vi "Dresden R2R Sputter 03.02.2018 IY24.vi"() -> ()   [LabVIEW 2009] (continued)
          }
        }
        n1372 = case shown="0, Default" w2342 {
          tunnel: w2348 -> [_ w2692 _]
          tunnel: w2349 -> [_ _ w2693]
          tunnel: [u32[][] [] ("24-bit pixmap") w2692 w2693] -> w2341
          frame #0 {
          }
          frame #1 {
          }
          frame #2 {
          }
        }
        n1373 = case shown="0, Default" w2339 {
          tunnel: w2348 -> [_ w2689 _]
          tunnel: w2349 -> [_ _ w2690]
          tunnel: [u32[][] [] ("24-bit pixmap") w2689 w2690] -> w2340
          frame #0 {
          }
          frame #1 {
          }
          frame #2 {
          }
        }
        n1374 = case shown="0, Default" w2327 {
          tunnel: w2348 -> [_ w2686 _]
          tunnel: w2349 -> [_ _ w2687]
          tunnel: [u32[][] [] ("24-bit pixmap") w2686 w2687] -> w2326
          frame #0 {
          }
          frame #1 {
          }
          frame #2 {
          }
        }
        n1375 = case shown="0, Default" w2323 {
          tunnel: w2348 -> [_ w2683 _]
          tunnel: w2349 -> [_ _ w2684]
          tunnel: [u32[][] [] ("24-bit pixmap") w2683 w2684] -> w2324
          frame #0 {
          }
          frame #1 {
          }
          frame #2 {
          }
        }
        n1376 = case shown="3" w2290 {
          tunnel: w2284 -> [_ w2679 _ _]
          tunnel: w2283 -> [_ _ w2680 _]
          tunnel: [u32[][] [] ("24-bit pixmap") w2679 w2680 w2681] -> w2291
          tunnel: w1979 -> [_ _ _ w2681]
          frame #0 {
          }
          frame #1 {
          }
          frame #2 {
          }
          frame #3 {
          }
        }
        n1377 = case shown="3" w2293 {
          tunnel: w2284 -> [_ w2675 _ _]
          tunnel: w2283 -> [_ _ w2676 _]
          tunnel: [u32[][] [] ("24-bit pixmap") w2675 w2676 w2677] -> w2292
          tunnel: w1979 -> [_ _ _ w2677]
          frame #0 {
          }
          frame #1 {
          }
          frame #2 {
          }
          frame #3 {
          }
        }
        n1378 = case shown="3" w2305 {
          tunnel: w2284 -> [_ w2671 _ _]
          tunnel: w2283 -> [_ _ w2672 _]
          tunnel: [u32[][] [] ("24-bit pixmap") w2671 w2672 w2673] -> w2306
          tunnel: w1979 -> [_ _ _ w2673]
          frame #0 {
          }
          frame #1 {
          }
          frame #2 {
          }
          frame #3 {
          }
        }
        n1379 = case shown="3" w2309 {
          tunnel: w2284 -> [_ w2667 _ _]
          tunnel: w2283 -> [_ _ w2668 _]
          tunnel: [u32[][] [] ("24-bit pixmap") w2667 w2668 w2669] -> w2308
          tunnel: w1979 -> [_ _ _ w2669]
          frame #0 {
          }
          frame #1 {
          }
          frame #2 {
          }
          frame #3 {
          }
        }
        n1380 = case shown="2" w2274 {
          tunnel: w2280 -> [_ w2664 _]
          tunnel: w2281 -> [_ _ w2665]
          tunnel: [u32[][] [] ("24-bit pixmap") w2664 w2665] -> w2273
          frame #0 {
          }
          frame #1 {
          }
          frame #2 {
          }
        }
        n1381 = case shown="2" w2271 {
          tunnel: w2280 -> [_ w2661 _]
          tunnel: w2281 -> [_ _ w2662]
          tunnel: [u32[][] [] ("24-bit pixmap") w2661 w2662] -> w2272
          frame #0 {
          }
          frame #1 {
          }
          frame #2 {
          }
        }
        n1382 = case shown="2" w2259 {
          tunnel: w2280 -> [_ w2658 _]
          tunnel: w2281 -> [_ _ w2659]
          tunnel: [u32[][] [] ("24-bit pixmap") w2658 w2659] -> w2258
          frame #0 {
          }
          frame #1 {
          }
          frame #2 {
          }
        }
        n1383 = case shown="2" w2255 {
          tunnel: w2280 -> [_ w2655 _]
          tunnel: w2281 -> [_ _ w2656]
          tunnel: [u32[][] [] ("24-bit pixmap") w2655 w2656] -> w2256
          frame #0 {
          }
          frame #1 {
          }
          frame #2 {
          }
        }
        n1384 = case shown="0, Default" w2222 {
          tunnel: w2216 -> [_ w2652 _]
          tunnel: w2215 -> [_ _ w2653]
          tunnel: [u32[][] [] ("24-bit pixmap") w2652 w2653] -> w2223
          frame #0 {
          }
          frame #1 {
          }
          frame #2 {
          }
        }
        n1385 = case shown="0, Default" w2225 {
          tunnel: w2216 -> [_ w2649 _]
          tunnel: w2215 -> [_ _ w2650]
          tunnel: [u32[][] [] ("24-bit pixmap") w2649 w2650] -> w2224
          frame #0 {
          }
          frame #1 {
          }
          frame #2 {
          }
        }
        n1386 = case shown="0, Default" w2237 {
          tunnel: w2216 -> [_ w2646 _]
          tunnel: w2215 -> [_ _ w2647]
          tunnel: [u32[][] [] ("24-bit pixmap") w2646 w2647] -> w2238
          frame #0 {
          }
          frame #1 {
          }
          frame #2 {
          }
        }
        n1387 = case shown="0, Default" w2241 {
          tunnel: w2216 -> [_ w2643 _]
          tunnel: w2215 -> [_ _ w2644]
          tunnel: [u32[][] [] ("24-bit pixmap") w2643 w2644] -> w2240
          frame #0 {
          }
          frame #1 {
          }
          frame #2 {
          }
        }
        n1388 = case shown="0, Default" w2206 {
          tunnel: w2212 -> [_ w2640 _]
          tunnel: w2213 -> [_ _ w2641]
          tunnel: [u32[][] [] ("24-bit pixmap") w2640 w2641] -> w2205
          frame #0 {
          }
          frame #1 {
          }
          frame #2 {
          }
        }
        n1389 = case shown="0, Default" w2203 {
          tunnel: w2212 -> [_ w2637 _]
          tunnel: w2213 -> [_ _ w2638]
          tunnel: [u32[][] [] ("24-bit pixmap") w2637 w2638] -> w2204
          frame #0 {
          }
          frame #1 {
          }
          frame #2 {
          }
        }
        n1390 = case shown="0, Default" w2191 {
          tunnel: w2212 -> [_ w2634 _]
          tunnel: w2213 -> [_ _ w2635]
          tunnel: [u32[][] [] ("24-bit pixmap") w2634 w2635] -> w2190
          frame #0 {
          }
          frame #1 {
          }
          frame #2 {
          }
        }
        n1391 = case shown="0, Default" w2154 {
          tunnel: w2148 -> [_ w2628 _]
          tunnel: w2147 -> [_ _ w2629]
          tunnel: [u32[][] [] ("24-bit pixmap") w2628 w2629] -> w2155
          frame #0 {
          }
          frame #1 {
          }
          frame #2 {
          }
        }
        n1392 = case shown="0, Default" w2187 {
          tunnel: w2212 -> [_ w2631 _]
          tunnel: w2213 -> [_ _ w2632]
          tunnel: [u32[][] [] ("24-bit pixmap") w2631 w2632] -> w2188
          frame #0 {
          }
          frame #1 {
          }
          frame #2 {
          }
        }
        n1393 = case shown="0, Default" w2157 {
          tunnel: w2148 -> [_ w2625 _]
          tunnel: w2147 -> [_ _ w2626]
          tunnel: [u32[][] [] ("24-bit pixmap") w2625 w2626] -> w2156
          frame #0 {
          }
          frame #1 {
          }
          frame #2 {
          }
        }
        n1394 = case shown="0, Default" w2169 {
          tunnel: w2148 -> [_ w2622 _]
          tunnel: w2147 -> [_ _ w2623]
          tunnel: [u32[][] [] ("24-bit pixmap") w2622 w2623] -> w2170
          frame #0 {
          }
          frame #1 {
          }
          frame #2 {
          }
        }
        n1395 = case shown="0, Default" w2141 {
          tunnel: w2066 -> [_ w2616 _]
          tunnel: w2118 -> [_ _ w2617]
          tunnel: [u32[][] [] ("24-bit pixmap") w2616 w2617] -> w2144
          frame #0 {
          }
          frame #1 {
          }
          frame #2 {
          }
        }
        n1396 = case shown="2" w2173 {
          tunnel: w2148 -> [_ w2619 _]
          tunnel: w2147 -> [_ _ w2620]
          tunnel: [u32[][] [] ("24-bit pixmap") w2619 w2620] -> w2172
          frame #0 {
          }
          frame #1 {
          }
          frame #2 {
          }
        }
        n1397 = case shown="2" w2131 {
          tunnel: w2066 -> [_ w2613 _]
          tunnel: w2118 -> [_ _ w2614]
          tunnel: [u32[][] [] ("24-bit pixmap") w2613 w2614] -> w2117
          frame #0 {
          }
          frame #1 {
          }
          frame #2 {
          }
        }
        n1398 = case shown="1" w2130 {
          tunnel: w2066 -> [_ w2610 _]
          tunnel: w2118 -> [_ _ w2611]
          tunnel: [u32[][] [] ("24-bit pixmap") w2610 w2611] -> w2116
          frame #0 {
          }
          frame #1 {
          }
          frame #2 {
          }
        }
        n1399 = case shown="2" w2129 {
          tunnel: w2066 -> [_ w2607 _]
          tunnel: w2118 -> [_ _ w2608]
          tunnel: [u32[][] [] ("24-bit pixmap") w2607 w2608] -> w2115
          frame #0 {
          }
          frame #1 {
          }
          frame #2 {
          }
        }
        n1400 = case shown="2" w2113 {
          tunnel: w2065 -> [_ w2604 _]
          tunnel: w2064 -> [_ _ w2605]
          tunnel: [u32[][] [] ("24-bit pixmap") w2604 w2605] -> w2114
          frame #0 {
          }
          frame #1 {
          }
          frame #2 {
          }
        }
        n1401 = case shown="2" w2108 {
          tunnel: w2065 -> [_ w2601 _]
          tunnel: w2064 -> [_ _ w2602]
          tunnel: [u32[][] [] ("24-bit pixmap") w2601 w2602] -> w2107
          frame #0 {
          }
          frame #1 {
          }
          frame #2 {
          }
        }
        n1402 = case shown="2" w2105 {
          tunnel: w2065 -> [_ w2598 _]
          tunnel: w2064 -> [_ _ w2599]
          tunnel: [u32[][] [] ("24-bit pixmap") w2598 w2599] -> w2106
          frame #0 {
          }
          frame #1 {
          }
          frame #2 {
          }
        }
        n1403 = case shown="2" w2100 {
          tunnel: w2063 -> [_ w2595 _]
          tunnel: w2062 -> [_ _ w2596]
          tunnel: [u32[][] [] ("24-bit pixmap") w2595 w2596] -> w2099
          frame #0 {
          }
          frame #1 {
          }
          frame #2 {
          }
        }
        n1404 = case shown="2" w2092 {
          tunnel: w2063 -> [_ w2589 _]
          tunnel: w2062 -> [_ _ w2590]
          tunnel: [u32[][] [] ("24-bit pixmap") w2589 w2590] -> w2091
          frame #0 {
          }
          frame #1 {
          }
          frame #2 {
          }
        }
        n1405 = case shown="2" w2097 {
          tunnel: w2063 -> [_ w2592 _]
          tunnel: w2062 -> [_ _ w2593]
          tunnel: [u32[][] [] ("24-bit pixmap") w2592 w2593] -> w2098
          frame #0 {
          }
          frame #1 {
          }
          frame #2 {
          }
        }
        n1406 = case shown="2" w2060 {
          tunnel: w2037 -> [_ w2586 _]
          tunnel: w2036 -> [_ _ w2587]
          tunnel: [u32[][] [] ("24-bit pixmap") w2586 w2587] -> w2061
          frame #0 {
          }
          frame #1 {
          }
          frame #2 {
          }
        }
        n1407 = case shown="2" w2055 {
          tunnel: w2037 -> [_ w2583 _]
          tunnel: w2036 -> [_ _ w2584]
          tunnel: [u32[][] [] ("24-bit pixmap") w2583 w2584] -> w2054
          frame #0 {
          }
          frame #1 {
          }
          frame #2 {
          }
        }
        n1408 = case shown="2" w2052 {
          tunnel: w2037 -> [_ w2580 _]
          tunnel: w2036 -> [_ _ w2581]
          tunnel: [u32[][] [] ("24-bit pixmap") w2580 w2581] -> w2053
          frame #0 {
          }
          frame #1 {
          }
          frame #2 {
          }
        }
        n1409 = case shown="2" w2033 {
          tunnel: w1989 -> [_ w2577 _]
          tunnel: w1988 -> [_ _ w2578]
          tunnel: [u32[][] [] ("24-bit pixmap") w2577 w2578] -> w2032
          frame #0 {
          }
          frame #1 {
          }
          frame #2 {
          }
        }
        n1410 = case shown="2" w2030 {
          tunnel: w1989 -> [_ w2574 _]
          tunnel: w1988 -> [_ _ w2575]
          tunnel: [u32[][] [] ("24-bit pixmap") w2574 w2575] -> w2031
          frame #0 {
          }
          frame #1 {
          }
          frame #2 {
          }
        }
        n1411 = case shown="2" w2025 {
          tunnel: w1989 -> [_ w2571 _]
          tunnel: w1988 -> [_ _ w2572]
          tunnel: [u32[][] [] ("24-bit pixmap") w2571 w2572] -> w2024
          frame #0 {
          }
          frame #1 {
          }
          frame #2 {
          }
        }
        n1412 = case shown="2" w2022 {
          tunnel: w1987 -> [_ w2568 _]
          tunnel: w1986 -> [_ _ w2569]
          tunnel: [u32[][] [] ("24-bit pixmap") w2568 w2569] -> w2023
          frame #0 {
          }
          frame #1 {
          }
          frame #2 {
          }
        }
        n1413 = case shown="2" w2017 {
          tunnel: w1987 -> [_ w2565 _]
          tunnel: w1986 -> [_ _ w2566]
          tunnel: [u32[][] [] ("24-bit pixmap") w2565 w2566] -> w2016
          frame #0 {
          }
          frame #1 {
          }
          frame #2 {
          }
        }
        n1414 = case shown="0, Default" w2014 {
          tunnel: w1987 -> [_ w2562 _]
          tunnel: w1986 -> [_ _ w2563]
          tunnel: [u32[][] [] ("24-bit pixmap") w2562 w2563] -> w2015
          frame #0 {
          }
          frame #1 {
          }
          frame #2 {
          }
        }
        n1415 = case shown="1" w1974 {
          tunnel: w1947 -> [_ w2560]
          tunnel: [u32[][] [] ("24-bit pixmap") w2560] -> w1971
          frame #0 {
          }
          frame #1 {
          }
        }
        n1416 = case shown="1" w1968 {
          tunnel: w1947 -> [_ w2558]
          tunnel: [u32[][] [] ("24-bit pixmap") w2558] -> w1970
          frame #0 {
          }
          frame #1 {
          }
        }
        n1417 = case shown="1" w1958 {
          tunnel: w1947 -> [_ w2556]
          tunnel: [u32[][] [] ("24-bit pixmap") w2556] -> w1956
          frame #0 {
          }
          frame #1 {
          }
        }
        n1418 = case shown="1" w1952 {
          tunnel: w1947 -> [_ w2554]
          tunnel: [u32[][] [] ("24-bit pixmap") w2554] -> w1954
          frame #0 {
          }
          frame #1 {
          }
        }
        n1419 = call-poly <vilib>:"Draw Unflattened Pixmap.vi"("data (RGB format)"=w1941) -> ("new picture"=w2546:picture)  [unwired: 8 in]
        n1420 = call-poly <vilib>:"Draw Unflattened Pixmap.vi"("picture"=w2546, "top left point(0, 0)"=cluster{"x":i16, "y":i16} {"x"=1103, "y"=31}, "data (RGB format)"=w2545) -> ("new picture"=w2537:picture)  [unwired: 6 in]
        n1421 = call-poly <vilib>:"Draw Unflattened Pixmap.vi"("picture"=w2537, "top left point(0, 0)"=cluster{"x":i16, "y":i16} {"x"=778, "y"=31}, "data (RGB format)"=w2544) -> ("new picture"=w2529:picture)  [unwired: 6 in]
        n1422 = call-poly <vilib>:"Draw Unflattened Pixmap.vi"("picture"=w2529, "top left point(0, 0)"=cluster{"x":i16, "y":i16} {"x"=453, "y"=31}, "data (RGB format)"=w2530) -> ("new picture"=w1940:picture)  [unwired: 6 in]
        n1423 = call-poly <vilib>:"Draw Unflattened Pixmap.vi"("picture"=w1940, "top left point(0, 0)"=cluster{"x":i16, "y":i16} {"x"=128, "y"=31}, "data (RGB format)"=w2528) -> ("new picture"=w2490:picture)  [unwired: 6 in]
        n1424 = call-poly <vilib>:"Draw Unflattened Pixmap.vi"("picture"=w2490, "top left point(0, 0)"=cluster{"x":i16, "y":i16} {"x"=1076, "y"=146} ("top left point(0, 0) 4"), "data (RGB format)"=w2497) -> ("new picture"=w2505:picture)  [unwired: 6 in]
        n1425 = call-poly <vilib>:"Draw Unflattened Pixmap.vi"("picture"=w2505, "top left point(0, 0)"=cluster{"x":i16, "y":i16} {"x"=751, "y"=146} ("top left point(0, 0) 3"), "data (RGB format)"=w2498) -> ("new picture"=w2513:picture)  [unwired: 6 in]
        n1426 = call-poly <vilib>:"Draw Unflattened Pixmap.vi"("picture"=w2513, "top left point(0, 0)"=cluster{"x":i16, "y":i16} {"x"=426, "y"=146} ("top left point(0, 0) 2"), "data (RGB format)"=w2512) -> ("new picture"=w2521:picture)  [unwired: 6 in]
        n1427 = call-poly <vilib>:"Draw Unflattened Pixmap.vi"("picture"=w2521, "top left point(0, 0)"=cluster{"x":i16, "y":i16} {"x"=100, "y"=146}, "data (RGB format)"=w2514) -> ("new picture"=w2452:picture)  [unwired: 6 in]
        n1428 = call-poly <vilib>:"Draw Unflattened Pixmap.vi"("picture"=w2452, "top left point(0, 0)"=cluster{"x":i16, "y":i16} {"x"=1181, "y"=150} ("top left point(0, 0) 4"), "data (RGB format)"=w2477) -> ("new picture"=w2469:picture)  [unwired: 6 in]
        n1429 = call-poly <vilib>:"Draw Unflattened Pixmap.vi"("picture"=w2469, "top left point(0, 0)"=cluster{"x":i16, "y":i16} {"x"=856, "y"=150} ("top left point(0, 0) 3"), "data (RGB format)"=w2476) -> ("new picture"=w2461:picture)  [unwired: 6 in]
        n1430 = call-poly <vilib>:"Draw Unflattened Pixmap.vi"("picture"=w2461, "top left point(0, 0)"=cluster{"x":i16, "y":i16} {"x"=531, "y"=150} ("top left point(0, 0) 2"), "data (RGB format)"=w2462) -> ("new picture"=w2453:picture)  [unwired: 6 in]
        n1431 = call-poly <vilib>:"Draw Unflattened Pixmap.vi"("picture"=w2453, "top left point(0, 0)"=cluster{"x":i16, "y":i16} {"x"=205, "y"=150}, "data (RGB format)"=w2460) -> ("new picture"=w2418:picture)  [unwired: 6 in]
        n1432 = call-poly <vilib>:"Draw Unflattened Pixmap.vi"("picture"=w2418, "top left point(0, 0)"=cluster{"x":i16, "y":i16} {"x"=1162, "y"=215} ("top left point(0, 0) 4"), "data (RGB format)"=w2427) -> ("new picture"=w2435:picture)  [unwired: 6 in]
        n1433 = call-poly <vilib>:"Draw Unflattened Pixmap.vi"("picture"=w2435, "top left point(0, 0)"=cluster{"x":i16, "y":i16} {"x"=838, "y"=215} ("top left point(0, 0) 3"), "data (RGB format)"=w2428) -> ("new picture"=w2443:picture)  [unwired: 6 in]
        n1434 = call-poly <vilib>:"Draw Unflattened Pixmap.vi"("picture"=w2443, "top left point(0, 0)"=cluster{"x":i16, "y":i16} {"x"=513, "y"=217} ("top left point(0, 0) 2"), "data (RGB format)"=w2442) -> ("new picture"=w2451:picture)  [unwired: 6 in]
        n1435 = call-poly <vilib>:"Draw Unflattened Pixmap.vi"("picture"=w2451, "top left point(0, 0)"=cluster{"x":i16, "y":i16} {"x"=187, "y"=215}, "data (RGB format)"=w2444) -> ("new picture"=w2384:picture)  [unwired: 6 in]
        n1436 = call-poly <vilib>:"Draw Unflattened Pixmap.vi"("picture"=w2384, "top left point(0, 0)"=cluster{"x":i16, "y":i16} {"x"=1120, "y"=323} ("top left point(0, 0) 4"), "data (RGB format)"=w2409) -> ("new picture"=w2401:picture)  [unwired: 6 in]
        n1437 = call-poly <vilib>:"Draw Unflattened Pixmap.vi"("picture"=w2401, "top left point(0, 0)"=cluster{"x":i16, "y":i16} {"x"=794, "y"=323} ("top left point(0, 0) 3"), "data (RGB format)"=w2408) -> ("new picture"=w2393:picture)  [unwired: 6 in]
        n1438 = call-poly <vilib>:"Draw Unflattened Pixmap.vi"("picture"=w2393, "top left point(0, 0)"=cluster{"x":i16, "y":i16} {"x"=468, "y"=323} ("top left point(0, 0) 2"), "data (RGB format)"=w2394) -> ("new picture"=w2385:picture)  [unwired: 6 in]
        n1439 = call-poly <vilib>:"Draw Unflattened Pixmap.vi"("picture"=w2385, "top left point(0, 0)"=cluster{"x":i16, "y":i16} {"x"=143, "y"=323}, "data (RGB format)"=w2392) -> ("new picture"=w2350:picture)  [unwired: 6 in]
        n1440 = call-poly <vilib>:"Draw Unflattened Pixmap.vi"("picture"=w2350, "top left point(0, 0)"=cluster{"x":i16, "y":i16} {"x"=1061, "y"=399} ("top left point(0, 0) 4"), "data (RGB format)"=w2359) -> ("new picture"=w2367:picture)  [unwired: 6 in]
        n1441 = call-poly <vilib>:"Draw Unflattened Pixmap.vi"("picture"=w2367, "top left point(0, 0)"=cluster{"x":i16, "y":i16} {"x"=735, "y"=399} ("top left point(0, 0) 3"), "data (RGB format)"=w2360) -> ("new picture"=w2375:picture)  [unwired: 6 in]
        n1442 = call-poly <vilib>:"Draw Unflattened Pixmap.vi"("picture"=w2375, "top left point(0, 0)"=cluster{"x":i16, "y":i16} {"x"=409, "y"=399} ("top left point(0, 0) 2"), "data (RGB format)"=w2374) -> ("new picture"=w2383:picture)  [unwired: 6 in]
        n1443 = call-poly <vilib>:"Draw Unflattened Pixmap.vi"("picture"=w2383, "top left point(0, 0)"=cluster{"x":i16, "y":i16} {"x"=83, "y"=399}, "data (RGB format)"=w2376) -> ("new picture"=w2316:picture)  [unwired: 6 in]
        n1444 = call-poly <vilib>:"Draw Unflattened Pixmap.vi"("picture"=w2316, "top left point(0, 0)"=cluster{"x":i16, "y":i16} {"x"=1117, "y"=399} ("top left point(0, 0) 4"), "data (RGB format)"=w2341) -> ("new picture"=w2333:picture)  [unwired: 6 in]
        n1445 = call-poly <vilib>:"Draw Unflattened Pixmap.vi"("picture"=w2333, "top left point(0, 0)"=cluster{"x":i16, "y":i16} {"x"=791, "y"=399} ("top left point(0, 0) 3"), "data (RGB format)"=w2340) -> ("new picture"=w2325:picture)  [unwired: 6 in]
        n1446 = call-poly <vilib>:"Draw Unflattened Pixmap.vi"("picture"=w2325, "top left point(0, 0)"=cluster{"x":i16, "y":i16} {"x"=465, "y"=399} ("top left point(0, 0) 2"), "data (RGB format)"=w2326) -> ("new picture"=w2317:picture)  [unwired: 6 in]
        n1447 = call-poly <vilib>:"Draw Unflattened Pixmap.vi"("picture"=w2317, "top left point(0, 0)"=cluster{"x":i16, "y":i16} {"x"=139, "y"=398}, "data (RGB format)"=w2324) -> ("new picture"=w2282:picture)  [unwired: 6 in]
        n1448 = call-poly <vilib>:"Draw Unflattened Pixmap.vi"("picture"=w2282, "top left point(0, 0)"=cluster{"x":i16, "y":i16} {"x"=1109, "y"=459} ("top left point(0, 0) 4"), "data (RGB format)"=w2291) -> ("new picture"=w2299:picture)  [unwired: 6 in]
        n1449 = call-poly <vilib>:"Draw Unflattened Pixmap.vi"("picture"=w2299, "top left point(0, 0)"=cluster{"x":i16, "y":i16} {"x"=783, "y"=459} ("top left point(0, 0) 3"), "data (RGB format)"=w2292) -> ("new picture"=w2307:picture)  [unwired: 6 in]
        n1450 = call-poly <vilib>:"Draw Unflattened Pixmap.vi"("picture"=w2307, "top left point(0, 0)"=cluster{"x":i16, "y":i16} {"x"=457, "y"=459} ("top left point(0, 0) 2"), "data (RGB format)"=w2306) -> ("new picture"=w2315:picture)  [unwired: 6 in]
        n1451 = call-poly <vilib>:"Draw Unflattened Pixmap.vi"("picture"=w2315, "top left point(0, 0)"=cluster{"x":i16, "y":i16} {"x"=131, "y"=459}, "data (RGB format)"=w2308) -> ("new picture"=w2248:picture)  [unwired: 6 in]
        n1452 = call-poly <vilib>:"Draw Unflattened Pixmap.vi"("picture"=w2248, "top left point(0, 0)"=cluster{"x":i16, "y":i16} {"x"=1038, "y"=701} ("top left point(0, 0) 4"), "data (RGB format)"=w2273) -> ("new picture"=w2265:picture)  [unwired: 6 in]
        n1453 = call-poly <vilib>:"Draw Unflattened Pixmap.vi"("picture"=w2265, "top left point(0, 0)"=cluster{"x":i16, "y":i16} {"x"=712, "y"=701} ("top left point(0, 0) 3"), "data (RGB format)"=w2272) -> ("new picture"=w2257:picture)  [unwired: 6 in]
        n1454 = call-poly <vilib>:"Draw Unflattened Pixmap.vi"("picture"=w2257, "top left point(0, 0)"=cluster{"x":i16, "y":i16} {"x"=386, "y"=701} ("top left point(0, 0) 2"), "data (RGB format)"=w2258) -> ("new picture"=w2249:picture)  [unwired: 6 in]
        n1455 = call-poly <vilib>:"Draw Unflattened Pixmap.vi"("picture"=w2249, "top left point(0, 0)"=cluster{"x":i16, "y":i16} {"x"=60, "y"=701}, "data (RGB format)"=w2256) -> ("new picture"=w2214:picture)  [unwired: 6 in]
        n1456 = call-poly <vilib>:"Draw Unflattened Pixmap.vi"("picture"=w2214, "top left point(0, 0)"=cluster{"x":i16, "y":i16} {"x"=1090, "y"=705} ("top left point(0, 0) 4"), "data (RGB format)"=w2223) -> ("new picture"=w2231:picture)  [unwired: 6 in]
        n1457 = call-poly <vilib>:"Draw Unflattened Pixmap.vi"("picture"=w2231, "top left point(0, 0)"=cluster{"x":i16, "y":i16} {"x"=765, "y"=705} ("top left point(0, 0) 3"), "data (RGB format)"=w2224) -> ("new picture"=w2239:picture)  [unwired: 6 in]
        n1458 = call-poly <vilib>:"Draw Unflattened Pixmap.vi"("picture"=w2239, "top left point(0, 0)"=cluster{"x":i16, "y":i16} {"x"=439, "y"=705} ("top left point(0, 0) 2"), "data (RGB format)"=w2238) -> ("new picture"=w2247:picture)  [unwired: 6 in]
        n1459 = call-poly <vilib>:"Draw Unflattened Pixmap.vi"("picture"=w2247, "top left point(0, 0)"=cluster{"x":i16, "y":i16} {"x"=113, "y"=705}, "data (RGB format)"=w2240) -> ("new picture"=w2180:picture)  [unwired: 6 in]
        n1460 = call-poly <vilib>:"Draw Unflattened Pixmap.vi"("picture"=w2180, "top left point(0, 0)"=cluster{"x":i16, "y":i16} {"x"=1152, "y"=717} ("top left point(0, 0) 4"), "data (RGB format)"=w2205) -> ("new picture"=w2197:picture)  [unwired: 6 in]
        n1461 = call-poly <vilib>:"Draw Unflattened Pixmap.vi"("picture"=w2197, "top left point(0, 0)"=cluster{"x":i16, "y":i16} {"x"=827, "y"=717} ("top left point(0, 0) 3"), "data (RGB format)"=w2204) -> ("new picture"=w2189:picture)  [unwired: 6 in]
        n1462 = call-poly <vilib>:"Draw Unflattened Pixmap.vi"("picture"=w2189, "top left point(0, 0)"=cluster{"x":i16, "y":i16} {"x"=501, "y"=717} ("top left point(0, 0) 2"), "data (RGB format)"=w2190) -> ("new picture"=w2181:picture)  [unwired: 6 in]
        n1463 = call-poly <vilib>:"Draw Unflattened Pixmap.vi"("picture"=w2181, "top left point(0, 0)"=cluster{"x":i16, "y":i16} {"x"=175, "y"=717}, "data (RGB format)"=w2188) -> ("new picture"=w2146:picture)  [unwired: 6 in]
        n1464 = call-poly <vilib>:"Draw Unflattened Pixmap.vi"("picture"=w2146, "top left point(0, 0)"=cluster{"x":i16, "y":i16} {"x"=1164, "y"=753} ("top left point(0, 0) 4"), "data (RGB format)"=w2155) -> ("new picture"=w2163:picture)  [unwired: 6 in]
        n1465 = call-poly <vilib>:"Draw Unflattened Pixmap.vi"("picture"=w2163, "top left point(0, 0)"=cluster{"x":i16, "y":i16} {"x"=838, "y"=753} ("top left point(0, 0) 3"), "data (RGB format)"=w2156) -> ("new picture"=w2171:picture)  [unwired: 6 in]
        n1466 = call-poly <vilib>:"Draw Unflattened Pixmap.vi"("picture"=w2171, "top left point(0, 0)"=cluster{"x":i16, "y":i16} {"x"=512, "y"=753} ("top left point(0, 0) 2"), "data (RGB format)"=w2170) -> ("new picture"=w2179:picture)  [unwired: 6 in]
        n1467 = call-poly <vilib>:"Draw Unflattened Pixmap.vi"("picture"=w2179, "top left point(0, 0)"=cluster{"x":i16, "y":i16} {"x"=186, "y"=753}, "data (RGB format)"=w2172) -> ("new picture"=w2145:picture)  [unwired: 6 in]
        n1468 = call-poly <vilib>:"Draw Unflattened Pixmap.vi"("picture"=w2145, "top left point(0, 0)"=cluster{"x":i16, "y":i16} {"x"=1238, "y"=723}, "data (RGB format)"=w2144) -> ("new picture"=w2126:picture)  [unwired: 6 in]
        n1469 = call-poly <vilib>:"Draw Unflattened Pixmap.vi"("picture"=w2126, "top left point(0, 0)"=cluster{"x":i16, "y":i16} {"x"=913, "y"=723}, "data (RGB format)"=w2117) -> ("new picture"=w2127:picture)  [unwired: 6 in]
        n1470 = call-poly <vilib>:"Draw Unflattened Pixmap.vi"("picture"=w2127, "top left point(0, 0)"=cluster{"x":i16, "y":i16} {"x"=587, "y"=723}, "data (RGB format)"=w2116) -> ("new picture"=w2128:picture)  [unwired: 6 in]
        n1471 = call-poly <vilib>:"Draw Unflattened Pixmap.vi"("picture"=w2128, "top left point(0, 0)"=cluster{"x":i16, "y":i16} {"x"=260, "y"=723}, "data (RGB format)"=w2115) -> ("new picture"=w2090:picture)  [unwired: 6 in]
        n1472 = call-poly <vilib>:"Draw Unflattened Pixmap.vi"("picture"=w2090, "top left point(0, 0)"=cluster{"x":i16, "y":i16} {"x"=1039, "y"=465}, "data (RGB format)"=w2114) -> ("new picture"=w2089:picture)  [unwired: 6 in]
        n1473 = call-poly <vilib>:"Draw Unflattened Pixmap.vi"("picture"=w2089, "top left point(0, 0)"=cluster{"x":i16, "y":i16} {"x"=713, "y"=465}, "data (RGB format)"=w2107) -> ("new picture"=w2088:picture)  [unwired: 6 in]
        n1474 = call-poly <vilib>:"Draw Unflattened Pixmap.vi"("picture"=w2088, "top left point(0, 0)"=cluster{"x":i16, "y":i16} {"x"=387, "y"=465}, "data (RGB format)"=w2106) -> ("new picture"=w2087:picture)  [unwired: 6 in]
        n1475 = call-poly <vilib>:"Draw Unflattened Pixmap.vi"("picture"=w2087, "top left point(0, 0)"=cluster{"x":i16, "y":i16} {"x"=883, "y"=467}, "data (RGB format)"=w2099) -> ("new picture"=w2086:picture)  [unwired: 6 in]
        n1476 = call-poly <vilib>:"Draw Unflattened Pixmap.vi"("picture"=w2086, "top left point(0, 0)"=cluster{"x":i16, "y":i16} {"x"=557, "y"=467}, "data (RGB format)"=w2098) -> ("new picture"=w2085:picture)  [unwired: 6 in]
        n1477 = call-poly <vilib>:"Draw Unflattened Pixmap.vi"("picture"=w2085, "top left point(0, 0)"=cluster{"x":i16, "y":i16} {"x"=232, "y"=467}, "data (RGB format)"=w2091) -> ("new picture"=w2039:picture)  [unwired: 6 in]
        n1478 = call-poly <vilib>:"Draw Unflattened Pixmap.vi"("picture"=w2039, "top left point(0, 0)"=cluster{"x":i16, "y":i16} {"x"=958, "y"=528}, "data (RGB format)"=w2061) -> ("new picture"=w2040:picture)  [unwired: 6 in]
        n1479 = call-poly <vilib>:"Draw Unflattened Pixmap.vi"("picture"=w2040, "top left point(0, 0)"=cluster{"x":i16, "y":i16} {"x"=633, "y"=528}, "data (RGB format)"=w2054) -> ("new picture"=w2038:picture)  [unwired: 6 in]
        n1480 = call-poly <vilib>:"Draw Unflattened Pixmap.vi"("picture"=w2038, "top left point(0, 0)"=cluster{"x":i16, "y":i16} {"x"=308, "y"=528}, "data (RGB format)"=w2053) -> ("new picture"=w2006:picture)  [unwired: 6 in]
        n1481 = call-poly <vilib>:"Draw Unflattened Pixmap.vi"("picture"=w2006, "top left point(0, 0)"=cluster{"x":i16, "y":i16} {"x"=985, "y"=263}, "data (RGB format)"=w2032) -> ("new picture"=w2007:picture)  [unwired: 6 in]
        n1482 = call-poly <vilib>:"Draw Unflattened Pixmap.vi"("picture"=w2007, "top left point(0, 0)"=cluster{"x":i16, "y":i16} {"x"=949, "y"=263}, "data (RGB format)"=w2031) -> ("new picture"=w2008:picture)  [unwired: 6 in]
        n1483 = call-poly <vilib>:"Draw Unflattened Pixmap.vi"("picture"=w2008, "top left point(0, 0)"=cluster{"x":i16, "y":i16} {"x"=660, "y"=263}, "data (RGB format)"=w2024) -> ("new picture"=w2009:picture)  [unwired: 6 in]
        n1484 = call-poly <vilib>:"Draw Unflattened Pixmap.vi"("picture"=w2009, "top left point(0, 0)"=cluster{"x":i16, "y":i16} {"x"=624, "y"=263}, "data (RGB format)"=w2023) -> ("new picture"=w2010:picture)  [unwired: 6 in]
        n1485 = call-poly <vilib>:"Draw Unflattened Pixmap.vi"("picture"=w2010, "top left point(0, 0)"=cluster{"x":i16, "y":i16} {"x"=334, "y"=263}, "data (RGB format)"=w2016) -> ("new picture"=w2011:picture)  [unwired: 6 in]
        n1486 = call-poly <vilib>:"Draw Unflattened Pixmap.vi"("picture"=w2011, "top left point(0, 0)"=cluster{"x":i16, "y":i16} {"x"=298, "y"=263}, "data (RGB format)"=w2015) -> ("new picture"=w1972:picture)  [unwired: 6 in]
        n1487 = call-poly <vilib>:"Draw Unflattened Pixmap.vi"("picture"=w1972, "top left point(0, 0)"=cluster{"x":i16, "y":i16} {"x"=58, "y"=545}, "data (RGB format)"=w1971) -> ("new picture"=w1963:picture)  [unwired: 6 in]
        n1488 = call-poly <vilib>:"Draw Unflattened Pixmap.vi"("picture"=w1963, "top left point(0, 0)"=cluster{"x":i16, "y":i16} {"x"=380, "y"=545}, "data (RGB format)"=w1970) -> ("new picture"=w1955:picture)  [unwired: 6 in]
        n1489 = call-poly <vilib>:"Draw Unflattened Pixmap.vi"("picture"=w1955, "top left point(0, 0)"=cluster{"x":i16, "y":i16} {"x"=705, "y"=545}, "data (RGB format)"=w1956) -> ("new picture"=w1946:picture)  [unwired: 6 in]
        n1490 = call-poly <vilib>:"Draw Unflattened Pixmap.vi"("picture"=w1946, "top left point(0, 0)"=cluster{"x":i16, "y":i16} {"x"=1033, "y"=545}, "data (RGB format)"=w1954) -> ("new picture"=w1945:picture)  [unwired: 6 in]
      }
      frame #1 {
        # "67"
        # "66"
        # "65"
        # "64"
        # "63"
        # "62"
        # "61"
        # "60"
        # "59"
        # "58"
        # "57"
        # "56"
        # "55"
        # "54"
        # "53"
        # "52"
        # "51"
        # "50"
        # "49"
        # "48"
        # "47"
        # "46"
        # "45"
        # "44"
        # "43"
        # "42"
        # "41"
        # "40"
        # "39"
        # "38"
        # "37"
        # "36"
        # "35"
        # "34"
        # "33"
        # "32"
        # "31"
        # "30"
        # "29"
        # "28"
        # "27"
        # "26"
        # "25"
        # "24"
        # "23"
        # "22"
        # "21"
        # "20"
        # "19"
        # "18"
        # "17"
        # "16"
        # "15"
        # "14"
        # "13"
        # "12"
        # "11"
        # "10"
        # "9"
        # "8"
        # "7"
        # "6"
        # "5"
        # "4"
        # "3"
        # "2"
        # "1"
        n1491 = property on="Background" class="Pict"() -> ("Mouse"=w3317:T37)  [unwired: 2 in, 2 out]
        n1492 = Unbundle(w3317) -> ("Mouse Position"=w3316:cluster{"X":i32, "Y":i32}, "Mouse Modifiers"=w3455:T38)
        "Mouse Position" <- w3316
        n1493 = Unbundle(w3316) -> ("X"=w2926:i32, "Y"=w2925:i32)
        n1494 = Unbundle(w3455) -> ("Button Down"=w3064:bool)  [unwired: 3 out]
        n1495 = In Range and Coerce(upper limit=197, x=w2925, lower limit=147) -> (In Range?=w3411:bool)  [unwired: 1 out]
        n1496 = In Range and Coerce(upper limit=197, x=w2925, lower limit=147) -> (In Range?=w3400:bool)  [unwired: 1 out]
        n1497 = In Range and Coerce(upper limit=126, x=w2926, lower limit=99) -> (In Range?=w3410:bool)  [unwired: 1 out]
        n1498 = In Range and Coerce(upper limit=774, x=w2926, lower limit=751) -> (In Range?=w3401:bool)  [unwired: 1 out]
        n1499 = In Range and Coerce(upper limit=197, x=w2925, lower limit=147) -> (In Range?=w3414:bool)  [unwired: 1 out]
        n1500 = In Range and Coerce(upper limit=743, x=w2925, lower limit=720) -> (In Range?=w3370:bool)  [unwired: 1 out]
        n1501 = In Range and Coerce(upper limit=197, x=w2925, lower limit=147) -> (In Range?=w3397:bool)  [unwired: 1 out]
        n1502 = In Range and Coerce(upper limit=446, x=w2926, lower limit=426) -> (In Range?=w3415:bool)  [unwired: 1 out]
        n1503 = In Range and Coerce(upper limit=743, x=w2925, lower limit=720) -> (In Range?=w3381:bool)  [unwired: 1 out]
        n1504 = In Range and Coerce(upper limit=213, x=w2926, lower limit=176) -> (In Range?=w3371:bool)  [unwired: 1 out]
        n1505 = In Range and Coerce(upper limit=1099, x=w2926, lower limit=1076) -> (In Range?=w3396:bool)  [unwired: 1 out]
        n1506 = In Range and Coerce(upper limit=863, x=w2926, lower limit=827) -> (In Range?=w3380:bool)  [unwired: 1 out]
        n1507 = In Range and Coerce(upper limit=347, x=w2925, lower limit=326) -> (In Range?=w3340:bool)  [unwired: 1 out]
        n1508 = In Range and Coerce(upper limit=306, x=w2926, lower limit=267) -> (In Range?=w2955:bool)  [unwired: 1 out]
        n1509 = In Range and Coerce(upper limit=758, x=w2925, lower limit=730) -> (In Range?=w2956:bool)  [unwired: 1 out]
        n1510 = In Range and Coerce(upper limit=633, x=w2926, lower limit=591) -> (In Range?=w2958:bool)  [unwired: 1 out]
        n1511 = In Range and Coerce(upper limit=758, x=w2925, lower limit=730) -> (In Range?=w2957:bool)  [unwired: 1 out]
        n1512 = In Range and Coerce(upper limit=961, x=w2926, lower limit=917) -> (In Range?=w2967:bool)  [unwired: 1 out]
        n1513 = In Range and Coerce(upper limit=758, x=w2925, lower limit=730) -> (In Range?=w2968:bool)  [unwired: 1 out]
        n1514 = In Range and Coerce(upper limit=1283, x=w2926, lower limit=1242) -> (In Range?=w2970:bool)  [unwired: 1 out]
        n1515 = In Range and Coerce(upper limit=758, x=w2925, lower limit=730) -> (In Range?=w2969:bool)  [unwired: 1 out]
        n1516 = In Range and Coerce(upper limit=115, x=w2925, lower limit=31) -> (In Range?=w3432:bool)  [unwired: 1 out]
        n1517 = In Range and Coerce(upper limit=743, x=w2925, lower limit=720) -> (In Range?=w3367:bool)  [unwired: 1 out]
        n1518 = In Range and Coerce(upper limit=347, x=w2925, lower limit=326) -> (In Range?=w3329:bool)  [unwired: 1 out]
        n1519 = In Range and Coerce(upper limit=182, x=w2926, lower limit=144) -> (In Range?=w3339:bool)  [unwired: 1 out]
        n1520 = In Range and Coerce(upper limit=450, x=w2925, lower limit=401) -> (In Range?=w3296:bool)  [unwired: 1 out]
        n1521 = In Range and Coerce(upper limit=456, x=w2925, lower limit=392) -> (In Range?=w3273:bool)  [unwired: 1 out]
        n1522 = In Range and Coerce(upper limit=685, x=w2925, lower limit=536) -> (In Range?=w3100:bool)  [unwired: 1 out]
        n1523 = In Range and Coerce(upper limit=751, x=w2925, lower limit=717) -> (In Range?=w3091:bool)  [unwired: 1 out]
        n1524 = In Range and Coerce(upper limit=212, x=w2926, lower limit=188) -> (In Range?=w2998:bool)  [unwired: 1 out]
        n1525 = In Range and Coerce(upper limit=789, x=w2925, lower limit=762) -> (In Range?=w2997:bool)  [unwired: 1 out]
        n1526 = In Range and Coerce(upper limit=538, x=w2926, lower limit=513) -> (In Range?=w2995:bool)  [unwired: 1 out]
        n1527 = In Range and Coerce(upper limit=789, x=w2925, lower limit=762) -> (In Range?=w2996:bool)  [unwired: 1 out]
        n1528 = In Range and Coerce(upper limit=863, x=w2926, lower limit=840) -> (In Range?=w2986:bool)  [unwired: 1 out]
        n1529 = In Range and Coerce(upper limit=789, x=w2925, lower limit=762) -> (In Range?=w2985:bool)  [unwired: 1 out]
        n1530 = In Range and Coerce(upper limit=1191, x=w2926, lower limit=1164) -> (In Range?=w2983:bool)  [unwired: 1 out]
        n1531 = In Range and Coerce(upper limit=789, x=w2925, lower limit=762) -> (In Range?=w2984:bool)  [unwired: 1 out]
        n1532 = In Range and Coerce(upper limit=85, x=w2926, lower limit=60) -> (In Range?=w2946:bool)  [unwired: 1 out]
        n1533 = In Range and Coerce(upper limit=735, x=w2925, lower limit=710) -> (In Range?=w2945:bool)  [unwired: 1 out]
        n1534 = In Range and Coerce(upper limit=408, x=w2926, lower limit=386) -> (In Range?=w2943:bool)  [unwired: 1 out]
        n1535 = In Range and Coerce(upper limit=735, x=w2925, lower limit=710) -> (In Range?=w2944:bool)  [unwired: 1 out]
        n1536 = In Range and Coerce(upper limit=738, x=w2926, lower limit=712) -> (In Range?=w2934:bool)  [unwired: 1 out]
        n1537 = In Range and Coerce(upper limit=735, x=w2925, lower limit=710) -> (In Range?=w2933:bool)  [unwired: 1 out]
        n1538 = In Range and Coerce(upper limit=1064, x=w2926, lower limit=1033) -> (In Range?=w2931:bool)  [unwired: 1 out]
        n1539 = In Range and Coerce(upper limit=735, x=w2925, lower limit=710) -> (In Range?=w2932:bool)  [unwired: 1 out]
        n1540 = In Range and Coerce(upper limit=115, x=w2925, lower limit=31) -> (In Range?=w3444:bool)  [unwired: 1 out]
        n1541 = In Range and Coerce(upper limit=212, x=w2926, lower limit=128) -> (In Range?=w3433:bool)  [unwired: 1 out]
        n1542 = In Range and Coerce(upper limit=742, x=w2925, lower limit=720) -> (In Range?=w3384:bool)  [unwired: 1 out]
        n1543 = In Range and Coerce(upper limit=539, x=w2926, lower limit=503) -> (In Range?=w3366:bool)  [unwired: 1 out]
        n1544 = In Range and Coerce(upper limit=832, x=w2926, lower limit=795) -> (In Range?=w3330:bool)  [unwired: 1 out]
        n1545 = In Range and Coerce(upper limit=450, x=w2925, lower limit=401) -> (In Range?=w3307:bool)  [unwired: 1 out]
        n1546 = In Range and Coerce(upper limit=107, x=w2926, lower limit=85) -> (In Range?=w3297:bool)  [unwired: 1 out]
        n1547 = In Range and Coerce(upper limit=456, x=w2925, lower limit=392) -> (In Range?=w3262:bool)  [unwired: 1 out]
        n1548 = In Range and Coerce(upper limit=211, x=w2926, lower limit=129) -> (In Range?=w3272:bool)  [unwired: 1 out]
        n1549 = In Range and Coerce(upper limit=296, x=w2925, lower limit=263) -> (In Range?=w3232:bool)  [unwired: 1 out]
        n1550 = In Range and Coerce(upper limit=492, x=w2925, lower limit=468) -> (In Range?=w3172:bool)  [unwired: 1 out]
        n1551 = In Range and Coerce(upper limit=485, x=w2925, lower limit=464) -> (In Range?=w3129:bool)  [unwired: 1 out]
        n1552 = In Range and Coerce(upper limit=351, x=w2926, lower limit=315) -> (In Range?=w3101:bool)  [unwired: 1 out]
        n1553 = In Range and Coerce(upper limit=751, x=w2925, lower limit=717) -> (In Range?=w3070:bool)  [unwired: 1 out]
        n1554 = In Range and Coerce(upper limit=149, x=w2926, lower limit=113) -> (In Range?=w3090:bool)  [unwired: 1 out]
        n1555 = In Range and Coerce(upper limit=239, x=w2926, lower limit=215) -> (In Range?=w3055:bool)  [unwired: 1 out]
        n1556 = In Range and Coerce(upper limit=178, x=w2925, lower limit=150) -> (In Range?=w3054:bool)  [unwired: 1 out]
        n1557 = In Range and Coerce(upper limit=566, x=w2926, lower limit=538) -> (In Range?=w3052:bool)  [unwired: 1 out]
        n1558 = In Range and Coerce(upper limit=178, x=w2925, lower limit=150) -> (In Range?=w3053:bool)  [unwired: 1 out]
        n1559 = In Range and Coerce(upper limit=894, x=w2926, lower limit=866) -> (In Range?=w3043:bool)  [unwired: 1 out]
        n1560 = In Range and Coerce(upper limit=178, x=w2925, lower limit=150) -> (In Range?=w3042:bool)  [unwired: 1 out]
        n1561 = In Range and Coerce(upper limit=1218, x=w2926, lower limit=1191) -> (In Range?=w3040:bool)  [unwired: 1 out]
        n1562 = In Range and Coerce(upper limit=178, x=w2925, lower limit=150) -> (In Range?=w3041:bool)  [unwired: 1 out]
        n1563 = In Range and Coerce(upper limit=221, x=w2926, lower limit=194) -> (In Range?=w3011:bool)  [unwired: 1 out]
        n1564 = In Range and Coerce(upper limit=259, x=w2925, lower limit=214) -> (In Range?=w3012:bool)  [unwired: 1 out]
        n1565 = In Range and Coerce(upper limit=547, x=w2926, lower limit=519) -> (In Range?=w3014:bool)  [unwired: 1 out]
        n1566 = In Range and Coerce(upper limit=259, x=w2925, lower limit=214) -> (In Range?=w3013:bool)  [unwired: 1 out]
        n1567 = In Range and Coerce(upper limit=873, x=w2926, lower limit=844) -> (In Range?=w3023:bool)  [unwired: 1 out]
        n1568 = In Range and Coerce(upper limit=259, x=w2925, lower limit=214) -> (In Range?=w3024:bool)  [unwired: 1 out]
        n1569 = In Range and Coerce(upper limit=1197, x=w2926, lower limit=1170) -> (In Range?=w3026:bool)  [unwired: 1 out]
        n1570 = In Range and Coerce(upper limit=259, x=w2925, lower limit=214) -> (In Range?=w3025:bool)  [unwired: 1 out]
        n1571 = In Range and Coerce(upper limit=867, x=w2926, lower limit=780) -> (In Range?=w3443:bool)  [unwired: 1 out]
        n1572 = In Range and Coerce(upper limit=1190, x=w2926, lower limit=1153) -> (In Range?=w3385:bool)  [unwired: 1 out]
        n1573 = In Range and Coerce(upper limit=347, x=w2925, lower limit=326) -> (In Range?=w3343:bool)  [unwired: 1 out]
        n1574 = In Range and Coerce(upper limit=759, x=w2926, lower limit=735) -> (In Range?=w3306:bool)  [unwired: 1 out]
        n1575 = In Range and Coerce(upper limit=861, x=w2926, lower limit=780) -> (In Range?=w3263:bool)  [unwired: 1 out]
        n1576 = In Range and Coerce(upper limit=296, x=w2925, lower limit=263) -> (In Range?=w3243:bool)  [unwired: 1 out]
        n1577 = In Range and Coerce(upper limit=357, x=w2926, lower limit=337) -> (In Range?=w3233:bool)  [unwired: 1 out]
        n1578 = In Range and Coerce(upper limit=298, x=w2925, lower limit=263) -> (In Range?=w3210:bool)  [unwired: 1 out]
        n1579 = In Range and Coerce(upper limit=492, x=w2925, lower limit=468) -> (In Range?=w3161:bool)  [unwired: 1 out]
        n1580 = In Range and Coerce(upper limit=919, x=w2926, lower limit=886) -> (In Range?=w3171:bool)  [unwired: 1 out]
        n1581 = In Range and Coerce(upper limit=492, x=w2925, lower limit=468) -> (In Range?=w3190:bool)  [unwired: 1 out]
        n1582 = In Range and Coerce(upper limit=485, x=w2925, lower limit=464) -> (In Range?=w3140:bool)  [unwired: 1 out]
        n1583 = In Range and Coerce(upper limit=225, x=w2926, lower limit=133) -> (In Range?=w3130:bool)  [unwired: 1 out]
        n1584 = In Range and Coerce(upper limit=685, x=w2925, lower limit=536) -> (In Range?=w3111:bool)  [unwired: 1 out]
        n1585 = In Range and Coerce(upper limit=1125, x=w2926, lower limit=1093) -> (In Range?=w3069:bool)  [unwired: 1 out]
        n1586 = In Range and Coerce(upper limit=751, x=w2925, lower limit=717) -> (In Range?=w3080:bool)  [unwired: 1 out]
        n1587 = In Range and Coerce(upper limit=115, x=w2925, lower limit=31) -> (In Range?=w3429:bool)  [unwired: 1 out]
        n1588 = In Range and Coerce(upper limit=347, x=w2925, lower limit=326) -> (In Range?=w3326:bool)  [unwired: 1 out]
        n1589 = In Range and Coerce(upper limit=506, x=w2926, lower limit=471) -> (In Range?=w3344:bool)  [unwired: 1 out]
        n1590 = In Range and Coerce(upper limit=450, x=w2925, lower limit=401) -> (In Range?=w3293:bool)  [unwired: 1 out]
        n1591 = In Range and Coerce(upper limit=456, x=w2925, lower limit=392) -> (In Range?=w3276:bool)  [unwired: 1 out]
        n1592 = In Range and Coerce(upper limit=652, x=w2926, lower limit=632) -> (In Range?=w3242:bool)  [unwired: 1 out]
        n1593 = In Range and Coerce(upper limit=1010, x=w2926, lower limit=988) -> (In Range?=w3209:bool)  [unwired: 1 out]
        n1594 = In Range and Coerce(upper limit=756, x=w2926, lower limit=716) -> (In Range?=w3162:bool)  [unwired: 1 out]
        n1595 = In Range and Coerce(upper limit=268, x=w2926, lower limit=235) -> (In Range?=w3191:bool)  [unwired: 1 out]
        n1596 = In Range and Coerce(upper limit=875, x=w2926, lower limit=783) -> (In Range?=w3139:bool)  [unwired: 1 out]